vi "UHR-Fleezers Control (host) - Avogadro v1.vi"() -> ()   [LabVIEW 2014] (continued)
          n911 = property on="Base N trap periods" class="DigNum (strict)"("Val(Sgnl)"=w1415) -> ()  [unwired: 2 in, 2 out]
        }
      }
    }
    frame #4 {
      # "Set FIFO size and run FPGA"
      n912 = local read "FPGA error out"() -> (w1417:errorcluster)
      n913 = xnode "Invoke Method"("FPGA VI Reference In"=w1418, "error in"=w1417, "Requested Depth"="Trap AI FIFO Depth") -> ("FPGA VI Reference Out"=w1422:T41, "error out"=w1423:errorcluster)  [unwired: 1 out]
      n914 = xnode "Invoke Method"("FPGA VI Reference In"=w1422, "error in"=w1423, "Requested Depth"="Trap Position FIFO Depth") -> ("FPGA VI Reference Out"=w1420:T41, "error out"=w1419:errorcluster)  [unwired: 1 out]
      n915 = xnode "Invoke Method"("FPGA VI Reference In"=w1420, "error in"=w1419) -> ("error out"=w1416:errorcluster)  [unwired: 1 in, 1 out]
      n916 = local write "FPGA error out"(w1416) -> ()
    }
    frame #5 {
      # "Adjust FPGA timing loop phases"
      n917 = flat-sequence "Initial FPGA Loop Relative Phase Adjustment" {
        tunnel: "Initial Phase Adjustment (AI1)" -> [w1457]
        tunnel: "Initial Phase Adjustment (GI)" -> [w1456]
        tunnel: "Initial Phase Adj. (MCL)" -> [w1455]
        tunnel: [w1458] -> w1442
        tunnel: [w1454] -> w1441
        tunnel: "Initial Phase Adjustment (APD Acq)" -> [w1453]
        tunnel: "Initial Phase Adjustment (APD 1 Gate)" -> [w1452]
        tunnel: "Initial Phase Adjustment (Green FB)" -> [w1451]
        tunnel: "Initial Phase Adjustment (GI) 2" -> [w1450]
        tunnel: "Initial Phase Adjustment (APD 2 Gate)" -> [w1449]
        tunnel: "Initial Phase Adjustment (RI)" -> [w1448]
        tunnel: "Initial Phase Adjustment (BI DO)" -> [w1447]
        tunnel: "Initial Phase Adjustment (BI AO)" -> [w1446]
        tunnel: "Initial Phase Adjustment (APD 3 Gate)" -> [w1445]
        tunnel: w1427 -> [w1444]
        tunnel: w1442 -> [w1460]
        tunnel: [w1461] -> w1440
        tunnel: w1441 -> [w1461]
        tunnel: [w1460] -> w1439
        tunnel: w1440 -> [w1465]
        tunnel: w1439 -> [w1464]
        tunnel: [w1462] -> w1426
        frame #0 {
          n918 = local read "FPGA error out"() -> (w1443:errorcluster)
          n919 = xnode "Read/Write Control"("FPGA VI Reference In"=w1444, "error in"=w1443, "Phase count adjustment"=w1457, "Phase count adjustment (GI)"=w1456, "Phase count adjustment (MCL)"=w1455, "Phase Count Adjustment (APD Acq)"=w1453, "Phase count adjustment (APD 1 Gate)"=w1452, "Phase count adjustment (APD 2 Gate)"=w1449, "Phase count adjustment (Green FB)"=w1451, "Phase count adjustment (GI) 2"=w1450, "Phase count adjustment (RI)"=w1448, "Phase count adjustment (BI AO)"=w1446, "Phase count adjustment (BI D)"=w1447, "Phase count adjustment (APD 3 Gate)"=w1445) -> ("FPGA VI Reference Out"=w1454:T41, "error out"=w1458:errorcluster)
        }
        frame #1 {
          n920 = Wait (ms)(milliseconds to wait=u32 100) -> ()  [unwired: 1 out]
        }
        frame #2 {
          w1463 = TRUE
          n921 = xnode "Read/Write Control"("FPGA VI Reference In"=w1465, "error in"=w1464, "+ phase"=w1463, "+ phase (GI)"=w1463, "+ phase (MCL)"=w1463, "+ phase (APD Acq)"=w1463, "+ phase (APD 1 Gate)"=w1463, "+ phase (APD 2 Gate)"=w1463, "+ phase (Green FB)"=w1463, "+ phase (GI) 2"=w1463, "+ phase (RI)"=w1463, "+ phase (BI AO)"=w1463, "+ phase (BI D)"=w1463, "+ phase (APD 3 Gate)"=w1463) -> ("error out"=w1462:errorcluster)  [unwired: 1 out]
        }
      }
      n922 = local write "FPGA error out"(w1426) -> ()
    }
    frame #6 {
      w1479 = 6.0  # clock mult.
      w1478 = 49152000.0  # TCXO frequ.
      w1483 = 6.0  # clock mult.
      w1484 = 49152000.0  # TCXO frequ.
      # "Added by ronen - definition of \nlimit frequencies when using dynamic feedback"
      # "Initialize trap RF synth board and set initial frequencies and amplitudes"
      n923 = local read "FPGA error out"() -> (w1493:errorcluster)
      n924 = call "Initialize RF boards - interlace 3.vi"("error in"=w1493, "FPGA VI Reference In"=w1494) -> ("error out"=w1495:errorcluster, "FPGA VI Reference Out"=w1515:T41)
      n925 = call "set RF board frequency - interlace.vi"("Board 2 Frequency Limits"=w1490, "Board 1 Frequency Limits"=w1471, "error in"=w1495, "FPGA VI Reference In"=w1515, "Board 2 Frequency 3 (MHz)"="BD 2 Frequency 3 (MHz)", "Board 1 Frequency 3 (MHz)"="BD 1 Frequency 3 (MHz)", "Board 2 Frequency 2 (MHz)"="BD 2 Frequency 2 (MHz)", "Board 2 Frequency 1 (MHz)"="BD 2 Frequency 1 (MHz)", "Board 1 Frequency 2 (MHz)"="BD 1 Frequency 2 (MHz)", "Board 1 Frequency 1  (MHz)"="BD 1 Frequency 1 (MHz)") -> ("error out"=w1498:errorcluster, "FPGA VI Reference Out"=w1470:T41)
      n926 = Unbundle By Name(w1471) -> ("Maximum"=w1481:dbl, "Minimum"=w1472:dbl)
      n927 = call "set RF board amplitude - interlace.vi"("Board 2 Amplitude Limits"=w1492, "Board 1 Amplitude Limits"=w1491, "error in"=w1498, "FPGA VI Reference In"=w1470, "Board 2 Amplitude 3 (%)"="BD 2 Amplitude 3 (%)", "Board 1 Amplitude 3 (%)"="BD 1 Amplitude 3 (%)", "Board 2 Amplitude 2 (%)"="BD 2 Amplitude 2 (%)", "Board 2 Amplitude 1 (%)"="BD 2 Amplitude 1 (%)", "Board 1 Amplitude 2 (%)"="BD 1 Amplitude 2 (%)", "Board 1 Amplitude 1 (%)"="BD 1 Amplitude 1 (%)") -> ("error out"=w1467:errorcluster)  [unwired: 1 out]
      n928 = Multiply(x=w1472, y=1000000.0) -> (x*y=w1476:dbl)
      n929 = Multiply(x=w1481, y=1000000.0) -> (x*y=w1486:dbl)
      n930 = Scale By Power Of 2(n=48, x=w1476) -> (x*2^n=w1474:dbl)
      n931 = Subtract(x="BD 1 Frequency 1 (MHz)", y="BD 1 Frequency 2 (MHz)") -> (x-y=w1505:dbl)
      n932 = Subtract(x="BD 2 Frequency 1 (MHz)", y="BD 2 Frequency 2 (MHz)") -> (x-y=w1506:dbl)
      n933 = Scale By Power Of 2(n=48, x=w1486) -> (x*2^n=w1488:dbl)
      n934 = Multiply(x=w1478, y=w1479) -> (x*y=w1480:dbl)
      n935 = Multiply(x=w1484, y=w1483) -> (x*y=w1482:dbl)
      n936 = Square(x=w1506) -> (x^2=w1508:dbl)
      n937 = Square(x=w1505) -> (x^2=w1507:dbl)
      n938 = Divide(x=w1474, y=w1480) -> (x/y=w1475:dbl)
      n939 = Divide(x=w1488, y=w1482) -> (x/y=w1487:dbl)
      n940 = Add(x=w1507, y=w1508) -> (x+y=w1509:dbl)
      n941 = To Unsigned Quad Integer(1:w1475) -> (0:w1468:u64)
      n942 = To Unsigned Quad Integer(1:w1487) -> (0:w1469:u64)
      n943 = Square Root(x=w1509) -> (sqrt(x)=w1510:dbl)
      n944 = local write "Trap Delta (MHz)"(w1510) -> ()
      n945 = xnode "Read/Write Control"("FPGA VI Reference In"=w1470, "error in"=w1467, "FB Max Frequency"=w1469, "FB Min frequency"=w1468) -> ("error out"=w1466:errorcluster)  [unwired: 1 out]
      n946 = local write "FPGA error out"(w1466) -> ()
    }
    frame #7 {
      n947 = local read "FPGA error out"() -> (w1517:errorcluster)
      n948 = flat-sequence {
        tunnel: [w1531] -> w1522
        tunnel: [w1530] -> w1521
        tunnel: w1518 -> [w1524]
        tunnel: w1517 -> [w1523]
        tunnel: [w1535] -> w1520
        tunnel: w1522 -> [w1535]
        tunnel: [w1534] -> w1519
        tunnel: w1521 -> [w1534]
        tunnel: w1520 -> [w1543]
        tunnel: w1519 -> [w1542]
        tunnel: [w1537] -> w1516
        frame #0 {
          n949 = xnode "Read/Write Control"("FPGA VI Reference In"=w1524, "error in"=w1523, "Direct RF Box  Communication"=FALSE) -> ("FPGA VI Reference Out"=w1531:T41, "error out"=w1530:errorcluster)
          n950 = local read "Trap 1 (ON/OFF)"() -> (w1525:bool)
          n951 = local write "Saving..."(FALSE ("Saving Data")) -> ()
          n952 = local write "Stop All"(FALSE ("Stop All")) -> ()
          n953 = local write "Index"(1.0 ("Index")) -> ()
          n954 = property on="Trap 1 ON" class="Bool (strict)"("Value"=w1525) -> ()  [unwired: 2 in, 2 out]
          "Manipulating Trap" <- FALSE ("Manipulating Trap")
        }
        frame #1 {
          n955 = local read "Trap 2 (ON/OFF)"() -> (w1533:bool)
          n956 = Wait (ms)(milliseconds to wait=u32 10) -> ()  [unwired: 1 out]
          n957 = property on="Trap 2 ON" class="Bool (strict)"("Val(Sgnl)"=w1533) -> ()  [unwired: 2 in, 2 out]
        }
        frame #2 {
          n958 = local read "Scan Range (nm)"() -> (w1538:dbl)
          n959 = xnode "Read/Write Control"("FPGA VI Reference In"=w1543, "error in"=w1542, "FPGA Controls  RF Box"=TRUE ("Direct RF Box  Communication")) -> ("error out"=w1537:errorcluster)  [unwired: 1 out]
          n960 = call "Update messages.vi"("Message to add"="UHR-Fleezers ready.", "Old message string"="") -> ("New message string"=w1541:string)
          n961 = local write "Messages"(w1541) -> ()
          n962 = property on="Scan Range (nm)" class="DigNum (strict)"("Val(Sgnl)"=w1538) -> ()  [unwired: 2 in, 2 out]
        }
      }
      n963 = local write "FPGA error out"(w1516) -> ()
    }
    frame #8 {
      w1577 = u32 0
      w1583 = cluster{u32, u32} {16777238, 16777238}
      w1578 = 0.0
      # "Initialize valves"
      # "Cursor control of trap\n3"
      # "Graph of positions and displacements in 2D"
      n964 = call "start_stage_trackball.vi"("Enum"=T38."Trackball XY", "Stage Controller port"=w1547) -> ("error out"=w1545:errorcluster)  [unwired: 1 in, 1 out]
      n965 = property on="Stage Control Serial Error" class="Clust (strict)"("Val(Sgnl)"=w1545) -> ()  [unwired: 2 in, 2 out]
      n966 = control-ref of="Positions \nand displacements"() -> (w1567:refnum<vi>)
      n967 = control-ref of="Piezo trap cursor control"() -> (w1579:refnum<vi>)
      n968 = property class="XYGraph (strict)"(reference=w1567, "XScale.Maximum"=6500.0, "XScale.Minimum"=-400.0, "YScale.Maximum"=400.0, "YScale.Minimum"=-3200.0, "Frame Color"=u32 9868950) -> (reference out=w1548:refnum<vi>)  [unwired: 1 in, 1 out]
      n969 = property class="XYGraph (strict)"(reference=w1548, "Active Plot"=0, "Plot.Plot Color"=u32 16711680, "Plot.Point Style"=2, "Plot.Line Width"=5, "Plot.Plot Interpolation"=0) -> (reference out=w1554:refnum<vi>)  [unwired: 1 in, 1 out]
      n970 = property class="XYGraph (strict)"(reference=w1579, "XScale.Maximum"=10.0, "XScale.Minimum"=w1578, "YScale.Maximum"=w1578, "YScale.Minimum"=-10.0, "Plot Area Colors"=w1583, "Frame Color"=u32 9868950, "XScale.GridColors"=w1583, "YScale.GridColors"=w1583, "Cursor.Cursor Color"=u32 16711680, "Active Cursor"=w1577, "Cursor.CursorMode"=w1577) -> ()  [unwired: 1 in, 2 out]
      n971 = property class="XYGraph (strict)"(reference=w1554, "Active Plot"=1, "Plot.Plot Color"=u32 16711680, "Plot.Point Style"=2, "Plot.Line Width"=5, "Plot.Plot Interpolation"=0) -> (reference out=w1555:refnum<vi>)  [unwired: 1 in, 1 out]
      n972 = property class="XYGraph (strict)"(reference=w1555, "Active Plot"=2, "Plot.Plot Color"=u32 16711680, "Plot.Point Style"=2, "Plot.Line Width"=5, "Plot.Plot Interpolation"=0) -> ()  [unwired: 1 in, 2 out]
      n973 = call "hamilton_controller.vi"("VISA resource name in"="Visa resource for valves", "action"=T42."CONNECT") -> ("error out"=w1576:errorcluster, "VISA resource name out"=w1573:refnum<visa-resource-name>)  [unwired: 8 in]
      n974 = call "hamilton_controller.vi"("VISA resource name in"=w1573, "error in"=w1576, "action"=T42."INITIALIZE VALVES") -> ("error out"=w1585:errorcluster)  [unwired: 7 in, 1 out]
    }
    frame #9 {
      # "Wait 5 s for all the event loops still being executed to finish."
      n975 = Wait (ms)(milliseconds to wait=u32 5000) -> ()  [unwired: 1 out]
      n976 = local read "FPGA error out"() -> (w1587:errorcluster)
    }
  }
  n977 = node-c288() -> (w34:T35)  [unwired: 4 out]
  n978 = disable-structure shown="Disabled" {
    frame Disabled {
      n979 = while "Duncan's play event loop" {
        stop <- w1591 stop-if-true
        n980 = Create User Event(user event datatype=TRUE ("Boolean")) -> (user event=w1592:refnum<user-event>)  [unwired: 1 in, 1 out]
        n981 = Create User Event(user event datatype=TRUE ("Boolean")) -> (user event=w1598:refnum<user-event>)  [unwired: 1 in, 1 out]
        n982 = global write "Global for fluorescence simulation mean (30 samples), (power series).vi" "Red Signal"(w1592) -> ()
        n983 = global write "Global for fluorescence simulation mean (30 samples), (power series).vi" "Green Signal"(w1598) -> ()
        n984 = register-events(w1598, w1592) -> (reference out=w1597:refnum<event-registration>)  [unwired: 2 in, 1 out]
        n985 = event shown="[1] \"Start assembly line\": Value Change" {
          selector: w1597 -> [_ _ _ _]
          dyn-events: _ -> [_ _ _ _]
          timeout: 100 -> [_ _ _ _]
          event Timeout {
            n986 = event-data() -> ()  [unwired: 1 in, 2 out]
          }
          event "Start assembly line": Value Change {
            n987 = event-data() -> ("OldVal"=w1600:bool)  [unwired: 1 in, 4 out]
            n988 = case shown="True" w1600 {
              selector: w1600 -> [_ w1601]
              frame False {
              }
              frame True {
                n989 = property on="Move to Position 3" class="Bool (strict)"("Val(Sgnl)"=w1601) -> ()  [unwired: 2 in, 2 out]
                n990 = case shown="1" "Numeric" {
                  frame 0, Default {
                  }
                  frame 1 {
                    n991 = property on="Green Laser ON" class="Bool (strict)"("Val(Sgnl)"=TRUE ("Value (Signaling)")) -> ()  [unwired: 2 in, 2 out]
                  }
                  frame 2 {
                    n992 = property on="Red Laser ON" class="Bool (strict)"("Val(Sgnl)"=TRUE) -> ()  [unwired: 2 in, 2 out]
                  }
                }
              }
            }
          }
          event User Event {
            n993 = event-data() -> ("Boolean"=w1605:bool)  [unwired: 1 in, 3 out]
            "Green Fluorophore" <- w1605
            n994 = property on="Start assembly line" class="Bool"("Val(Sgnl)"=w1605) -> ()  [unwired: 2 in, 2 out]
          }
          event User Event {
            n995 = event-data() -> ("Boolean"=w1606:bool)  [unwired: 1 in, 3 out]
            "Red Fluorophore" <- w1606
            n996 = property on="Start assembly line" class="Bool"("Val(Sgnl)"=w1606) -> ()  [unwired: 2 in, 2 out]
          }
        }
        n997 = property on="Get Fluorophore" class="Bool (strict)"("Val(Sgnl)"="Get Fluorophore") -> ()  [unwired: 2 in, 2 out]
        n998 = Wait (ms)(milliseconds to wait=u32 100) -> ()  [unwired: 1 out]
        n999 = local read "Stop All"() -> (w1590:bool)
        n1000 = Or(x=w1590, y="stop") -> (x .or. y?=w1591:bool)
      }
    }
    frame Enabled {
    }
  }
  n1001 = timed-loop "Rough control of MCL mirror stage (debugging)" {
    tunnel: [w1609] -> w74
    timing: w34 -> [_]
    timing-out: [_] -> w33
    tunnel: w25 -> [w1607]
    stop <- w1609 stop-if-true
    n1002 = node-c288() -> ()  [unwired: 2 out]
    n1003 = case shown="1" "MCL Mode" {
      tunnel: w1607 -> [_ w1612 w1659]
      frame 0, Default {
      }
      frame 1 {
        n1004 = node-c288() -> (w1614:T35)  [unwired: 4 out]
        n1005 = timed-loop "Oscillate MCL mirror" {
          timing: w1614 -> [_]
          timing-out: [_] -> w1613
          tunnel: w1612 -> [w1615]
          i -> [w1653]
          stop <- w1616 stop-if-true
          n1006 = node-c288() -> (w1652:i64)  [unwired: 1 out]
          n1007 = Multiply(x="AO1", y=32767.0) -> (x*y=w1648:dbl)
          n1008 = Multiply(x="AO2", y=32767.0) -> (x*y=w1643:dbl)
          n1009 = Divide(x=w1648, y=10.0) -> (x/y=w1649:dbl)
          n1010 = Divide(x=w1643, y=10.0) -> (x/y=w1644:dbl)
          n1011 = To Word Integer(number=w1649) -> (16bit integer=w1641:i16)
          n1012 = To Word Integer(number=w1644) -> (16bit integer=w1640:i16)
          n1013 = Divide(x=w1652, y=i64 1000) -> (x/y=w1623:dbl)
          n1014 = Multiply(x=w1623, y=w1653) -> (x*y=w1634:dbl)
          n1015 = Multiply(x="Osc. freq. (Hz) 2", y=6.283185307179586) -> (x*y=w1635:dbl)
          n1016 = Multiply(x=w1635, y=w1634) -> (x*y=w1633:dbl)
          n1017 = Sine(x=w1633) -> (sin(x)=w1632:dbl)
          n1018 = Multiply(x=w1632, y="Osc. amp. (V)") -> (x*y=w1630:dbl)
          n1019 = Add(x=w1630, y="Osc. center (V)") -> (x+y=w1628:dbl)
          n1020 = Divide(x=w1628, y=10.0) -> (x/y=w1626:dbl)
          n1021 = Multiply(x=w1626, y=32767.0) -> (x*y=w1621:dbl)
          n1022 = Select(t=w1621, s="Scan axis", f=w1641) -> (s? t:f=w1639:dbl)
          n1023 = Select(t=w1640, s="Scan axis", f=w1621) -> (s? t:f=w1638:dbl)
          n1024 = local read "MCL Mode"() -> (w1620:u16)
          n1025 = Not Equal?(x=w1620, y=u16 1) -> (x != y?=w1617:bool)
          n1026 = local read "Stop All"() -> (w1618:bool)
          n1027 = xnode "Read/Write Control"("FPGA VI Reference In"=w1615, "AO1 (Y)"=w1639, "AO2 (X)"=w1638) -> ()  [unwired: 1 in, 2 out]
          n1028 = Compound Arithmetic op=OR(w1618, w1617) -> (w1616:bool)
          n1029 = node-c288() -> ()  [unwired: 2 out]
        }
        n1030 = node-c288(w1613) -> ()  [unwired: 1 out]
      }
      frame 2 {
        n1031 = case shown="True" "Start Scan" {
          tunnel: w1659 -> [_ w1661]
          frame False {
          }
          frame True {
            n1032 = Subtract(x="End (V)", y="Begin (V)") -> (x-y=w1668:dbl)
            n1033 = Decrement(x="N Points") -> (x-1=w1667:dbl)
            n1034 = Divide(x=w1668, y=w1667) -> (x/y=w1665:dbl)
            n1035 = for {
              N: "N Points" -> [_]
              tunnel: "Begin (V)" -> [w1684]
              tunnel: [w1676] -> w1671 mode=indexing
              tunnel: w1665 -> [w1675]
              tunnel: [w1673] -> w1664 mode=indexing
              tunnel: w1661 -> [w1672]
              i -> [w1683]
              n1036 = Multiply(x=w1675, y=w1683) -> (x*y=w1682:dbl)
              n1037 = Add(x=w1684, y=w1682) -> (x+y=w1679:dbl)
              n1038 = local read "Scan axis"() -> (w1674:bool)
              n1039 = local read "AO1"() -> (w1681:dbl)
              n1040 = local read "AO2"() -> (w1680:dbl)
              n1041 = Select(t=w1679, s=w1674, f=w1681) -> (s? t:f=w1678:dbl)
              n1042 = Select(t=w1680, s=w1674, f=w1679) -> (s? t:f=w1677:dbl)
              n1043 = flat-sequence {
                tunnel: w1678 -> [w1688]
                tunnel: w1677 -> [w1687]
                tunnel: w1672 -> [w1685]
                tunnel: [w1698] -> w1676
                tunnel: [w1697] -> w1673
                frame #0 {
                  w1691 = 10.0 ("y")
                  w1686 = 32767.0 ("y")
                  n1044 = Multiply(x=w1688, y=w1686) -> (x*y=w1694:dbl)
                  n1045 = Multiply(x=w1687, y=w1686) -> (x*y=w1692:dbl)
                  n1046 = Divide(x=w1694, y=w1691) -> (x/y=w1695:dbl)
                  n1047 = Divide(x=w1692, y=w1691) -> (x/y=w1693:dbl)
                  n1048 = To Word Integer(number=w1695) -> (16bit integer=w1689:i16)
                  n1049 = To Word Integer(number=w1693) -> (16bit integer=w1690:i16)
                  n1050 = xnode "Read/Write Control"("FPGA VI Reference In"=w1685, "AO1 (Y)"=w1689, "AO2 (X)"=w1690) -> ()  [unwired: 1 in, 2 out]
                }
                frame #1 {
                  n1051 = Wait (ms)(milliseconds to wait="DAQ Delay (ms)") -> ()  [unwired: 1 out]
                }
                frame #2 {
                  n1052 = local read "Slow mean"() -> (w1698:dbl)
                  n1053 = local read "Sigma"() -> (w1697:dbl)
                }
              }
            }
            n1054 = Bundle("Begin (V)"="Begin (V)", w1665, w1671) -> (→"MCL Scan":cluster{"Begin (V)":dbl, dbl, dbl[]})  [unwired: 1 out]
            n1055 = Bundle("Begin (V)"="Begin (V)", w1665, w1664) -> (→"MCL Scan 2":cluster{"Begin (V)":dbl, dbl, dbl[]})  [unwired: 1 out]
          }
        }
      }
    }
    n1056 = local read "Stop All"() -> (w1609:bool)
    n1057 = node-c288() -> ()  [unwired: 2 out]
  }
  n1058 = node-c288(2 ("Processor")) -> (w65:T35)  [unwired: 3 out]
  n1059 = timed-loop "Basic control parameters (all FPGA settings, other basic controls)" {
    shift-right: [w1706] -> _
    shift-left: errorcluster {"status"=FALSE, "code"=0, "source"=""} ("error out") -> [_]
    tunnel: [w1705] -> _
    timing: w65 -> [_]
    timing-out: [_] -> w64
    tunnel: w47 -> [w1704]
    tunnel: w43 -> [w1703]
    tunnel: w42 -> [w1702]
    tunnel: w41 -> [w1701]
    tunnel: w40 -> [w1700]
    tunnel: w25 -> [w1699]
    stop <- w1705 stop-if-true
    n1060 = node-c288() -> ()  [unwired: 2 out]
    n1061 = event shown="[13] \"Load parameters\": Value Change" {
      selector: _ -> [_ _ _ _ _ _ _ _ _ _ _ _ _ _ _ _ _ _ _ _ _ _ _ _ _ _ _ _ _ _ _ _ _ _ _ _ _ _ _ _ _ _ _ _ _ _ _ _ _ _ _ _ _ _ _ _ _ _ _ _ _ _ _ _ _ _ _ _ _ _ _ _ _ _ _ _ _ _ _ _ _ _ _ _ _ _]
      dyn-events: _ -> [_ _ _ _ _ _ _ _ _ _ _ _ _ _ _ _ _ _ _ _ _ _ _ _ _ _ _ _ _ _ _ _ _ _ _ _ _ _ _ _ _ _ _ _ _ _ _ _ _ _ _ _ _ _ _ _ _ _ _ _ _ _ _ _ _ _ _ _ _ _ _ _ _ _ _ _ _ _ _ _ _ _ _ _ _ _]
      timeout: _ -> [_ _ _ _ _ _ _ _ _ _ _ _ _ _ _ _ _ _ _ _ _ _ _ _ _ _ _ _ _ _ _ _ _ _ _ _ _ _ _ _ _ _ _ _ _ _ _ _ _ _ _ _ _ _ _ _ _ _ _ _ _ _ _ _ _ _ _ _ _ _ _ _ _ _ _ _ _ _ _ _ _ _ _ _ _ _]
      tunnel: [w1746 _ _ _ w1773 _ _ _ _ _ _ _ w1879 _ _ w1966 w1968 w1975 w1977 w2047 _ w2089 w2115 w2143 w2168 w2195 w2221 w2250 _ w2255 w2349 w2353 w2390 _ w2475 w2478 w2481 w2491 w2494 _ w2501 _ _ _ _ _ _ _ _ _ _ _ _ _ _ _ _ _ _ _ w2996 _ _ _ _ w3033 _ _ _ _ _ _ _ _ _ _ _ _ _ _ _ _ _ _ _ _] -> w1706
      tunnel: [_ _ _ _ _ _ _ _ _ _ w1858 _ _ _ _ _ _ _ _ _ _ _ _ _ _ _ _ _ _ _ _ _ _ _ _ _ _ _ _ _ _ _ _ _ _ _ _ _ _ _ _ _ _ _ _ _ _ _ _ _ _ _ _ _ _ _ _ _ _ _ _ _ _ _ _ _ _ _ _ _ _ _ _ _ _ _] -> w1705
      tunnel: [_ _ _ _ _ _ _ _ "Round T1 X" _ _ _ _ _ _ _ _ _ _ _ _ _ _ _ _ _ _ _ _ _ _ _ _ _ _ _ _ _ _ _ _ _ _ _ _ _ _ _ _ _ _ _ _ _ _ _ _ _ _ _ _ _ _ _ _ _ _ _ _ _ _ _ _ _ _ _ _ _ _ _ _ _ _ _ _ _] -> _
      tunnel: [_ _ _ "Adjust Scale\nto Mean" _ _ _ _ _ _ _ _ _ _ _ _ _ _ _ _ _ _ _ _ _ _ _ _ _ "Test ttrig" _ _ _ _ _ _ _ _ _ _ _ _ _ _ _ _ _ _ _ _ w2743 w2807 w2854 w2903 _ _ _ _ _ _ _ _ _ _ _ _ _ _ _ _ _ _ _ _ _ _ _ _ _ _ _ _ _ _ _ _] -> _
      tunnel: [_ _ _ _ _ _ _ _ _ "Round T2 X" _ "Delayed Interlace Start" _ _ _ _ _ _ _ _ _ _ _ _ _ _ _ _ _ _ _ _ _ _ _ _ _ _ _ _ _ _ _ _ _ _ _ _ _ _ _ _ _ _ _ _ _ _ _ _ _ _ _ _ _ _ _ _ _ _ _ _ _ _ _ _ _ _ _ _ _ _ _ _ _ _] -> _
      tunnel: w1704 -> [_ _ _ _ _ _ _ _ _ _ _ _ _ _ _ _ _ _ _ _ _ _ _ _ _ _ _ _ _ _ _ _ _ _ _ _ _ _ _ _ _ _ _ _ _ _ w2713 w2721 w2728 w2734 w2742 _ _ w2902 _ _ _ _ _ _ _ _ _ _ _ _ _ _ _ _ _ _ _ _ _ _ _ _ _ _ _ _ _ _ _ _]
      tunnel: w1703 -> [_ _ _ _ _ _ _ _ _ _ _ _ _ _ _ _ _ _ _ _ _ _ _ _ _ _ _ _ _ _ _ _ _ _ _ _ _ _ _ _ _ _ _ _ w2600 _ _ _ _ _ _ w2806 _ _ w2909 _ w2921 _ w2937 _ _ _ _ _ _ _ _ _ _ _ _ _ _ _ _ _ _ _ _ _ _ _ _ _ _ _]
      tunnel: w1702 -> [_ _ _ _ _ _ _ _ _ _ _ _ _ _ _ _ _ _ _ _ _ _ _ _ _ _ _ _ _ _ _ _ _ _ _ _ _ _ _ _ _ _ _ _ _ _ _ _ _ _ _ _ _ _ _ _ _ _ _ _ _ _ _ _ _ _ _ _ _ _ _ _ _ _ _ _ _ _ _ _ _ _ _ _ _ _]
      tunnel: w1701 -> [_ _ _ _ _ _ _ _ _ _ _ _ _ _ _ _ _ _ _ _ _ _ _ _ _ _ _ _ _ _ _ _ _ _ _ _ _ _ _ _ _ w2512 _ _ _ _ _ _ _ _ _ _ w2853 _ _ w2915 _ w2929 _ w2963 _ _ _ _ _ _ _ _ _ _ _ _ _ _ _ _ _ _ _ _ _ _ _ _ _ _]
      tunnel: w1700 -> [_ _ _ _ _ _ _ _ _ _ _ _ _ _ _ _ _ _ _ _ _ _ _ _ _ _ _ _ _ _ _ _ _ _ _ _ _ _ _ _ _ _ _ _ _ _ _ _ _ _ _ _ _ _ _ _ _ _ _ _ _ _ _ _ _ _ _ _ _ _ _ _ _ _ _ _ _ _ _ _ _ _ _ _ _ _]
      tunnel: w1699 -> [w1709 _ _ _ w1772 _ w1798 _ _ _ _ _ w1870 _ _ w1950 w1967 w1974 w1976 w2012 _ w2078 w2113 w2125 w2150 w2178 w2198 w2226 w2251 w2253 w2257 w2350 w2354 _ w2472 w2476 w2479 w2489 w2492 _ w2500 _ _ _ _ _ _ _ _ _ _ _ _ _ _ _ _ _ _ _ w2989 _ w3010 _ w3017 w3032 _ w3039 w3066 w3073 w3089 w3097 _ w3108 _ w3152 _ _ w3206 w3237 w3241 w3249 _ w3313 w3323 w3342]
      tunnel: [_ _ _ _ _ _ _ _ _ _ w1857 _ _ _ _ _ _ _ _ _ _ _ _ _ _ _ _ _ _ _ _ _ _ _ _ _ _ _ _ _ _ _ w2592 w2596 _ _ _ _ _ _ _ _ _ _ _ _ _ _ _ _ _ _ _ _ _ _ _ _ _ _ _ _ _ _ _ _ _ _ _ _ _ _ _ _ _ _] -> _
      event "AI Count (ticks)", "Sets to FIFO (Traps)", "Save ave N", "FPGA Ave.", "# Samples/channel", "N sets to save": Value Change {
        # "RG 18-01-16 Increased amount of elements to read for trap position, to add x and y for piezo trap"
        # "So that if 'Save ave N' is updated, the AOD scanning code updates too."
        n1062 = event-data() -> ()  [unwired: 6 out]
        n1063 = local read "AI Count (ticks)"() -> (w1730:u16)
        n1064 = Divide(x=40000000.0, y=w1730) -> (x/y=w1722:dbl)
        "AI rate (Hz)" <- w1722
        "Ave. Rate (Hz)" <- w1722
        n1065 = Reciprocal(x=w1722) -> (1/x=→"Ave. Period (s)":dbl)
        n1066 = Unbundle By Name("Sets to FIFO (Traps)") -> ("Set 1"=w1713:bool, "Set 2"=w1712:bool, "Set 3"=w1711:bool)
        n1067 = Divide(x=w1722, y="N Acq Sets (Traps + Fl.)") -> (x/y=w1743:dbl)
        "Data Rate (Hz)" <- w1743
        n1068 = Reciprocal(x=w1743) -> (1/x=→"Data Period (s)":dbl)
        n1069 = Boolean To (0,1)(Boolean="Sets to FIFO (Traps)") -> (0, 1=w1738:cluster{"Set 1":i16, "Set 2":i16, "Set 3":i16})
        n1070 = xnode "Read/Write Control"("FPGA VI Reference In"=w1709, "ai count"=w1730, "Set 1"=w1713, "Set 2"=w1712, "Set 3"=w1711, "N of AI1 Int Acq Sets"="N Acq Sets (Traps + Fl.)") -> ("error out"=w1746:errorcluster)  [unwired: 1 in, 1 out]
        n1071 = Cluster To Array(cluster=w1738) -> (array=w1737:i16[])
        n1072 = local read "Save ave N"() -> (w1742:dbl)
        n1073 = To Unsigned Long Integer(number=w1737) -> (unsigned 32bit integer=w1719:u32[])
        n1074 = local read "Scan steps (AOD)"() -> (w1739:u64)
        n1075 = Multiply(x=w1730, y="N Acq Sets (Traps + Fl.)") -> (x*y=w1728:u16)
        n1076 = Add Array Elements(numeric array=w1719) -> (sum=w1731:u32)
        "Trap Sets" <- w1731
        n1077 = Divide(x=w1743, y=w1742) -> (x/y=w1741:dbl)
        "Save Data Rate (Hz)" <- w1741
        n1078 = Reciprocal(x=w1741) -> (1/x=→"Save Data Period (s)":dbl)
        n1079 = property on="Scan steps (AOD)" class="DigNum (strict)"("Val(Sgnl)"=w1739) -> ()  [unwired: 2 in, 2 out]
        n1080 = Multiply(x=w1728, y="# Samples/trap") -> (x*y=w1726:u32)
        "Counts/DMA" <- w1726
        n1081 = property on="Trap Disp. Downsample" class="DigNum (strict)"("Maximum"="# Samples/trap") -> ()  [unwired: 2 in, 2 out]
        n1082 = Multiply(x=w1731, y="# Samples/trap") -> (x*y=w1720:u32)
        "# Samples/channel" <- w1720
        n1083 = Multiply(x=w1720, y=u32 8) -> (x*y=→"Trap AI Elements/DMA read":u32)
        n1084 = local read "APD Int. Count"() -> (w1727:u32)
        n1085 = Multiply(x=w1720, y=u32 5) -> (x*y=→"Trap Pos Elements/DMA read":u32)
        n1086 = Divide(x=w1726, y=w1727) -> (x/y=w1717:dbl)
        "APD Samples/FIFO Acq." <- w1717
        n1087 = Divide(x=w1726, y=40000000.0) -> (x/y=w1724:dbl)
        "DMA Update Period (s)" <- w1724
        n1088 = local read "Number of APDs"() -> (w1710:u8)
        n1089 = Multiply(x=w1710, y=w1717) -> (x*y=→"APD Elements/DMA read":dbl)
        n1090 = property on="APD Disp. Downsample" class="DigNum (strict)"("Maximum"=w1717) -> ()  [unwired: 2 in, 2 out]
        n1091 = local read "N sets to save"() -> (w1736:u32)
        n1092 = Multiply(x=w1724, y=w1736) -> (x*y=→"Total Time (s) 2":dbl)
        "FPGA Averaging" <- FALSE ("FPGA Averaging")
      }
      event "Remove Offset": Value Change {
        n1093 = event-data() -> ()  [unwired: 7 out]
        n1094 = local write "Remove Offset"(FALSE ("Remove Offset")) -> ()
        n1095 = local read "Bead Mean (nm)"() -> (w1748:dbl)
        n1096 = local read "Offset (nm)"() -> (w1749:dbl)
        n1097 = Add(x=w1748, y=w1749) -> (x+y=w1747:dbl)
        n1098 = local write "Offset (nm)"(w1747) -> ()
      }
      event "Detector Type": Value Change {
        n1099 = event-data() -> ()  [unwired: 7 out]
        n1100 = local read "AI labels"() -> (w1753:string[])
        n1101 = property on="High Res. Display" class="Ring (strict)"("Strings []"=w1753) -> ()  [unwired: 2 in, 2 out]
        n1102 = Build Array (concatenate)(w1753, "none") -> (w1754:string[])
        n1103 = property on="FFT 1 Choice 1" class="Ring (strict)"("Strings []"=w1754) -> ()  [unwired: 2 in, 2 out]
        n1104 = property on="FFT 1 Choice 2" class="Ring (strict)"("Strings []"=w1754) -> ()  [unwired: 2 in, 2 out]
        n1105 = property on="FFT 2 Choice 1" class="Ring (strict)"("Strings []"=w1754) -> ()  [unwired: 2 in, 2 out]
        n1106 = property on="FFT 2 Choice 2" class="Ring (strict)"("Strings []"=w1754) -> ()  [unwired: 2 in, 2 out]
        n1107 = Bundle("APD 1", "APD 2", "APD 3") -> (w1757:cluster{string, string, string})  [unwired: 1 out]
        n1108 = Cluster To Array(cluster=w1757) -> (array=w1755:string[])
        n1109 = Build Array (concatenate)(w1755, w1754) -> (w1759:string[])
        n1110 = Array Size(array=w1759) -> (size(s)=w1751:i32)
        n1111 = property on="Signals to Plot" class="LstBox (strict)"("Item Names"=w1759) -> ()  [unwired: 2 in, 2 out]
        n1112 = property on="Signals to Plot" class="LstBox (strict)"("Number of Rows"=w1751) -> ()  [unwired: 2 in, 2 out]
        n1113 = property on="All Signals" class="WFChart (strict)"("LegNumRows"=w1751) -> ()  [unwired: 2 in, 2 out]
      }
      event "Adjust Scale\nto Mean": Value Change {
        n1114 = event-data() -> ()  [unwired: 7 out]
        n1115 = local read "APD rates cluster"() -> (w1762:T1)
        n1116 = Unbundle By Name(w1762) -> ("APD 1 Rate (Hz)"=w1761:dbl)
        n1117 = Multiply(x=1000.0, y="Above (kHz)") -> (x*y=w1768:dbl)
        n1118 = Multiply(x=1000.0, y="Below (kHz)") -> (x*y=w1766:dbl)
        n1119 = Add(x=w1768, y=w1761) -> (x+y=w1763:dbl)
        n1120 = Subtract(x=w1761, y=w1766) -> (x-y=w1764:dbl)
        n1121 = property on="APD Chart" class="WFChart (strict)"("YScale.Minimum"=w1764) -> ()  [unwired: 2 in, 2 out]
        n1122 = property on="APD Chart" class="WFChart (strict)"("YScale.Maximum"=w1763) -> ()  [unwired: 2 in, 2 out]
      }
      event "Phase adj. (AI1)", "+ phase (AI1)", "- phase (AI1)": Value Change {
        n1123 = event-data() -> ()  [unwired: 7 out]
        n1124 = Negate(x="Phase adj. (AI1)") -> (-x=w1780:i16)
        n1125 = Select(t=w1780, s="- phase (AI1)", f="Phase adj. (AI1)") -> (s? t:f=w1779:i16)
        n1126 = xnode "Read/Write Control"("FPGA VI Reference In"=w1772, "Phase count adjustment"=w1779) -> ("FPGA VI Reference Out"=w1778:T41, "error out"=w1777:errorcluster)  [unwired: 2 in]
        n1127 = Or(x="- phase (AI1)", y="+ phase (AI1)") -> (x .or. y?=w1774:bool)
        n1128 = xnode "Read/Write Control"("FPGA VI Reference In"=w1778, "error in"=w1777, "+ phase"=w1774) -> ("error out"=w1773:errorcluster)  [unwired: 1 in, 1 out]
      }
      event "Signals to Plot": Double Click {
        w1792 = u32 9868950 ("Color Box")
        n1129 = event-data() -> ("Row"=w1783:i32)  [unwired: 9 out]
        n1130 = property on="All Signals" class="WFChart (strict)"("Active Plot"=w1783) -> (error out=w1782:errorcluster)  [unwired: 2 in, 1 out]
        n1131 = property on="All Signals" class="WFChart (strict)" props=["Plot", "Plot Color", "Plot", "Visible?"](error in=w1782) -> (error out=w1785:errorcluster, "Plot.Visible?"=w1784:bool)  [unwired: 1 in, 2 out]
        n1132 = Select(t=FALSE ("Plot.Visible"), s=w1784, f=TRUE ("Plot.Visible")) -> (s? t:f=w1787:bool)
        n1133 = property on="All Signals" class="WFChart (strict)"(error in=w1785, "Plot.Visible?"=w1787) -> (error out=w1786:errorcluster)  [unwired: 1 in, 1 out]
        n1134 = property on="All Signals" class="WFChart (strict)"(error in=w1786) -> (error out=w1788:errorcluster, "Plot.Plot Color"=w1789:u32)  [unwired: 1 in, 1 out]
        n1135 = property on="Signals to Plot" class="LstBox (strict)"(error in=w1788, "Active Row"=w1783) -> (error out=w1793:errorcluster)  [unwired: 1 in, 1 out]
        n1136 = Select(t=w1789, s=w1787, f=u32 0) -> (s? t:f=w1794:u32)
        n1137 = property on="Signals to Plot" class="LstBox (strict)"(error in=w1793, "CellFontColor"=w1794, "SelColor"=w1792, "CellBG"=w1792, "CellFontSize"=u32 20 ("Active Row:Cell Font:Size"), "CellFontBold"=TRUE ("Active Row:Cell Font:Bold")) -> ()  [unwired: 1 in, 2 out]
      }
      event "BD 1 Frequency 1 (MHz)", "BD 1 Frequency 2 (MHz)", "BD 1 Frequency 3 (MHz)", "BD 2 Frequency 1 (MHz)", "BD 2 Frequency 2 (MHz)", "BD 2 Frequency 3 (MHz)", "Trap Delta (MHz)", "Update all trap values": Value Change {
        # "This is so you can set trap frequencies\nvia local variables and then update\nall at once"
        n1138 = event-data() -> ("CtlRef"=w1802:refnum<vi>)  [unwired: 6 out]
        n1139 = control-ref of="Trap Delta (MHz)"() -> (w1801:refnum<vi>)
        n1140 = Equal?(x=w1801, y=w1802) -> (x = y?=w1800:bool)
        n1141 = local write "Update all trap values"(FALSE ("Update all trap values")) -> ()
        n1142 = case shown="False" "Oscillate Set 1" {
          tunnel: w1800 -> [w1816 _]
          tunnel: w1798 -> [w1814 _]
          frame False {
            n1143 = local read "BD 1 Frequency 2 (MHz)"() -> (w1812:dbl)
            n1144 = case shown="False" "Symmetric?" {
              tunnel: "Trap Delta (MHz)" -> [w1838 w1845]
              tunnel: [w1839 w1843] -> w1804
              tunnel: [w1837 w1840] -> w1806
              tunnel: w1812 -> [w1839 _]
              frame False {
                n1145 = Subtract(x=w1839, y=w1838) -> (x-y=w1837:dbl)
              }
              frame True {
                w1842 = 75
                n1146 = Divide(x=w1845, y=2.0) -> (x/y=w1841:dbl)
                n1147 = Add(x=w1841, y=w1842) -> (x+y=w1843:dbl)
                n1148 = Subtract(x=w1842, y=w1841) -> (x-y=w1840:dbl)
              }
            }
            n1149 = local read "BD 1 Frequency 1 (MHz)"() -> (w1807:dbl)
            n1150 = Not(x="Symmetric?") -> (.not. x?=w1810:bool)
            n1151 = And(x=w1810, y="move Con X?") -> (x .and. y?=w1808:bool)
            n1152 = Subtract(x=w1807, y=w1806) -> (x-y=w1805:dbl)
            n1153 = Select(t=w1806, s=w1816, f=w1807) -> (s? t:f=w1815:dbl)
            n1154 = local read "Y RF Frequency Limits (MHz)"() -> (w1817:T23)
            n1155 = case shown="True" w1808 {
              tunnel: w1805 -> [_ w1836]
              frame False {
              }
              frame True {
                n1156 = property on="AOM X Cal (nm/MHz)" class="DigNum (strict)"() -> ("Value"=w1835:dbl)  [unwired: 2 in, 2 out]
                n1157 = property on="MCL Step Position Ratio" class="DigNum (strict)"() -> ("Value"=w1829:dbl)  [unwired: 2 in, 2 out]
                n1158 = Compound Arithmetic op=MULTIPLY(w1836, w1835, w1829) -> (w1834:dbl)
                n1159 = property on="MCL X Cal (nm/V)" class="DigNum (strict)"() -> ("Value"=w1833:dbl)  [unwired: 2 in, 2 out]
                n1160 = Divide(x=w1834, y=w1833) -> (x/y=w1832:dbl)
                n1161 = property on="AO2" class="Slide (strict)"() -> ("Value"=w1831:dbl)  [unwired: 2 in, 2 out]
                n1162 = Add(x=w1832, y=w1831) -> (x+y=w1830:dbl)
                n1163 = property on="AO2" class="Slide (strict)"("Val(Sgnl)"=w1830) -> ()  [unwired: 2 in, 2 out]
              }
            }
            n1164 = local read "X RF Frequency Limits (MHz)"() -> (w1818:T23)
            n1165 = local write "BD 1 Frequency 1 (MHz)"(w1815) -> ()
            n1166 = local read "BD 1 Frequency 3 (MHz)"() -> (w1827:dbl)
            n1167 = local read "BD 2 Frequency 1 (MHz)"() -> (w1821:dbl)
            n1168 = local read "BD 2 Frequency 2 (MHz)"() -> (w1820:dbl)
            n1169 = local read "BD 2 Frequency 3 (MHz)"() -> (w1828:dbl)
            n1170 = call "set RF board frequency - interlace.vi"("Board 2 Frequency Limits"=w1817, "Board 1 Frequency Limits"=w1818, "FPGA VI Reference In"=w1814, "Board 2 Frequency 3 (MHz)"=w1828, "Board 1 Frequency 3 (MHz)"=w1827, "Board 2 Frequency 2 (MHz)"=w1820, "Board 2 Frequency 1 (MHz)"=w1821, "Board 1 Frequency 2 (MHz)"=w1804, "Board 1 Frequency 1  (MHz)"=w1815) -> ()  [unwired: 1 in, 2 out]
            n1171 = Subtract(x=w1821, y=w1820) -> (x-y=w1825:dbl)
            n1172 = local write "BD 1 Frequency 2 (MHz)"(w1804) -> ()
            n1173 = Subtract(x=w1815, y=w1804) -> (x-y=w1826:dbl)
            n1174 = Square(x=w1825) -> (x^2=w1823:dbl)
            n1175 = Square(x=w1826) -> (x^2=w1824:dbl)
            n1176 = Add(x=w1824, y=w1823) -> (x+y=w1822:dbl)
            n1177 = Square Root(x=w1822) -> (sqrt(x)=w1819:dbl)
            n1178 = property on="Initial delta (MHz)" class="DigNum (strict)"("Val(Sgnl)"=w1819) -> ()  [unwired: 2 in, 2 out]
            n1179 = local write "Trap Delta (MHz)"(w1819) -> ()
          }
          frame True {
          }
        }
      }
      event "manual raster set": Value Change {
        n1180 = event-data() -> ()  [unwired: 7 out]
        n1181 = flat-sequence {
          frame #0 {
            n1182 = Replace Array Subset(array=u32[] [0] ("Index Values"), new element="manual raster set", index=0) -> (w1846:u32[])
            n1183 = property on="Saved AOD Raster Scan Parameter Sets" class="Arr (strict)"("Index Values"=w1846) -> ()  [unwired: 2 in, 2 out]
          }
          frame #1 {
            n1184 = property on="Load parameters" class="Bool (strict)"("Val(Sgnl)"=TRUE ("Value (Signaling)")) -> ()  [unwired: 2 in, 2 out]
          }
        }
      }
      event "Round T1 X": Value Change {
        n1185 = event-data() -> ()  [unwired: 7 out]
        n1186 = local read "BD 1 Frequency 1 (MHz)"() -> (w1853:dbl)
        n1187 = Round To Nearest(number=w1853) -> (nearest integer value=w1852:dbl)
        n1188 = property on="BD 1 Frequency 1 (MHz)" class="DigNum (strict)"("Val(Sgnl)"=w1852) -> ()  [unwired: 2 in, 2 out]
      }
      event "Round T2 X": Value Change {
        n1189 = event-data() -> ()  [unwired: 7 out]
        n1190 = local read "BD 1 Frequency 2 (MHz)"() -> (w1855:dbl)
        n1191 = Round To Nearest(number=w1855) -> (nearest integer value=w1854:dbl)
        n1192 = property on="BD 1 Frequency 2 (MHz)" class="DigNum (strict)"("Val(Sgnl)"=w1854) -> ()  [unwired: 2 in, 2 out]
      }
      event "Stop All": Value Change {
        n1193 = event-data() -> ()  [unwired: 7 out]
        n1194 = flat-sequence {
          tunnel: [w1861] -> w1859
          tunnel: [w1864] -> w1857
          tunnel: w1859 -> [w1864]
          tunnel: [TRUE] -> w1858
          frame #0 {
            n1195 = local read "Visa resource for valves"() -> (w1860:refnum<visa-resource-name>)
            n1196 = call "hamilton_controller.vi"("VISA resource name in"=w1860, "action"=T42."DISCONNECT") -> ("error out"=w1861:errorcluster)  [unwired: 8 in, 1 out]
          }
          frame #1 {
          }
        }
      }
      event "Delayed Interlace Start": Value Change {
        n1197 = event-data() -> ()  [unwired: 7 out]
        n1198 = flat-sequence {
          frame #0 {
            n1199 = Multiply(x="Delay to Interlace (s)", y=1000.0) -> (x*y=w1866:dbl)
            n1200 = Wait (ms)(milliseconds to wait=w1866) -> ()  [unwired: 1 out]
          }
          frame #1 {
            n1201 = property on="Laser interlacing mode" class="RadioBtnsControl (strict)"("Val(Sgnl)"=enum32{"Laser ON", "Laser OFF", "Interlace"}."Interlace" ("Value (Signaling)")) -> ()  [unwired: 2 in, 2 out]
          }
        }
      }
      event "BD 1 Amplitude 1 (%)", "BD 1 Amplitude 2 (%)", "BD 1 Amplitude 3 (%)", "BD 2 Amplitude 1 (%)", "BD 2 Amplitude 2 (%)", "BD 2 Amplitude 3 (%)", "Trap 1 ON", "Trap 2 ON", "Trap 3 ON", "Feedback On/Off", "All FB On/Off": Value Change {
        w1891 = i16 1 ("f")
        n1202 = event-data() -> ()  [unwired: 7 out]
        n1203 = local write "Trap 1 (ON/OFF)"("Trap 1 ON") -> ()
        n1204 = local write "Trap 2 (ON/OFF)"("Trap 2 ON") -> ()
        n1205 = Boolean To (0,1)(Boolean="Trap 3 ON") -> (0, 1=w1892:i16)
        n1206 = Boolean To (0,1)(Boolean="Trap 1 ON") -> (0, 1=w1893:i16)
        n1207 = Boolean To (0,1)(Boolean="Trap 2 ON") -> (0, 1=w1894:i16)
        n1208 = Select(t=w1894, s="Trap ON/OFF X or Y Amp?", f=w1891) -> (s? t:f=w1889:i16)
        n1209 = Select(t=w1893, s="Trap ON/OFF X or Y Amp?", f=w1891) -> (s? t:f=w1890:i16)
        n1210 = Select(t=w1892, s="Trap ON/OFF X or Y Amp?", f=w1891) -> (s? t:f=w1888:i16)
        n1211 = Select(t=w1891, s="Trap ON/OFF X or Y Amp?", f=w1894) -> (s? t:f=w1886:i16)
        n1212 = Select(t=w1891, s="Trap ON/OFF X or Y Amp?", f=w1893) -> (s? t:f=w1887:i16)
        n1213 = Select(t=w1891, s="Trap ON/OFF X or Y Amp?", f=w1892) -> (s? t:f=w1885:i16)
        n1214 = And(x="All FB On/Off", y="Feedback On/Off") -> (x .and. y?=w1883:cluster{"Set 1":bool, "Set 2":bool})
        n1215 = local read "BD 1 Amplitude 1 (%)"() -> (w1901:dbl)
        n1216 = local read "BD 1 Amplitude 2 (%)"() -> (w1900:dbl)
        n1217 = local read "BD 1 Amplitude 3 (%)"() -> (w1899:dbl)
        n1218 = Unbundle By Name(w1883) -> ("Set 1"=w1878:bool, "Set 2"=w1875:bool)
        n1219 = local read "Y RF Amplitude Limits (%)"() -> (w1871:T23)
        n1220 = local read "X RF Amplitude Limits (%)"() -> (w1872:T23)
        n1221 = local read "BD 2 Amplitude 1 (%)"() -> (w1902:dbl)
        n1222 = local read "BD 2 Amplitude 2 (%)"() -> (w1903:dbl)
        n1223 = local read "BD 2 Amplitude 3 (%)"() -> (w1904:dbl)
        n1224 = And(x="Trap 2 ON", y=w1875) -> (x .and. y?=w1873:bool)
        n1225 = And(x="Trap 1 ON", y=w1878) -> (x .and. y?=w1876:bool)
        n1226 = Multiply(x=w1890, y=w1901) -> (x*y=w1898:dbl)
        n1227 = Multiply(x=w1900, y=w1889) -> (x*y=w1896:dbl)
        n1228 = Multiply(x=w1899, y=w1888) -> (x*y=w1897:dbl)
        n1229 = Multiply(x=w1902, y=w1887) -> (x*y=w1905:dbl)
        n1230 = Multiply(x=w1903, y=w1886) -> (x*y=w1906:dbl)
        n1231 = Multiply(x=w1904, y=w1885) -> (x*y=w1907:dbl)
        n1232 = call "set RF board amplitude - interlace.vi"("Board 2 Amplitude Limits"=w1871, "Board 1 Amplitude Limits"=w1872, "FPGA VI Reference In"=w1870, "Board 2 Amplitude 3 (%)"=w1907, "Board 1 Amplitude 3 (%)"=w1897, "Board 2 Amplitude 2 (%)"=w1906, "Board 2 Amplitude 1 (%)"=w1905, "Board 1 Amplitude 2 (%)"=w1896, "Board 1 Amplitude 1 (%)"=w1898) -> ("error out"=w1880:errorcluster, "FPGA VI Reference Out"=w1881:T41)  [unwired: 1 in]
        n1233 = xnode "Read/Write Control"("FPGA VI Reference In"=w1881, "error in"=w1880, "FB On/Off Set 1"=w1876, "FB On/Off Set 2"=w1873) -> ("error out"=w1879:errorcluster)  [unwired: 1 out]
      }
      event "Load parameters": Value Change {
        n1234 = event-data() -> ()  [unwired: 7 out]
        n1235 = property on="Saved AOD Raster Scan Parameter Sets" class="Arr (strict)"() -> ("Index Values"=w1918:u32[])  [unwired: 2 in, 2 out]
        n1236 = Index Array(array=w1918, index=0) -> (element=w1915:u32)
        n1237 = local write "Load parameters"(FALSE ("Load parameters")) -> ()
        n1238 = Index Array(array="Saved AOD Raster Scan Parameter Sets", index=w1915) -> (element=w1914:T46)
        n1239 = Unbundle By Name(w1914) -> ("Scan Range AOD (nm) 2"=w1913:dbl, "Step Size AOD (nm) 2"=w1912:dbl, "Scan Speed AOD (nm/s) 2"=w1911:dbl, "Number of scans (AOD) 2"=w1910:u16)
        n1240 = flat-sequence {
          tunnel: w1913 -> [w1921]
          tunnel: w1912 -> [w1920]
          tunnel: w1911 -> [w1919]
          tunnel: w1910 -> [w1922]
          frame #0 {
            n1241 = local write "Scan Speed (nm/s)"(w1919) -> ()
            n1242 = local write "Scan Range (nm)"(w1921) -> ()
            n1243 = local write "Step Size (nm)"(w1920) -> ()
          }
          frame #1 {
            n1244 = property on="Number of F/B Scans (AOD)" class="DigNum (strict)"("Val(Sgnl)"=w1922) -> ()  [unwired: 2 in, 2 out]
          }
        }
      }
      event "Trap 1 (ON/OFF)", "Trap 2 (ON/OFF)": Value Change {
        n1245 = event-data() -> ()  [unwired: 7 out]
        n1246 = flat-sequence {
          tunnel: [w1932] -> w1927
          tunnel: w1927 -> [w1947]
          tunnel: [w1933] -> w1923
          frame #0 {
            n1247 = local read "Trap 1 ON"() -> (w1932:bool)
          }
          frame #1 {
            n1248 = Exclusive Or(1:w1947, 2:"Trap 1 (ON/OFF)") -> (0:w1940:bool)
            n1249 = Select(t="on", s="Trap 2 (ON/OFF)", f="off") -> (s? t:f=w1939:string)
            n1250 = Select(t="on", s="Trap 1 (ON/OFF)", f="off") -> (s? t:f=w1935:string)
            n1251 = Build Array("trap 1 ", w1935) -> (w1934:string[])
            n1252 = Build Array("trap 2 " ("f"), w1939) -> (w1937:string[])
            n1253 = Select(t=w1934, s=w1940, f=w1937) -> (s? t:f=w1933:string[])
            n1254 = property on="Trap 1 ON" class="Bool (strict)"("Val(Sgnl)"="Trap 1 (ON/OFF)") -> ()  [unwired: 2 in, 2 out]
            n1255 = property on="Trap 2 ON" class="Bool (strict)"("Val(Sgnl)"="Trap 2 (ON/OFF)") -> ()  [unwired: 2 in, 2 out]
          }
        }
        n1256 = local read "Saving..."() -> (w1926:bool)
        n1257 = local read "Save Event Log?"() -> (w1925:bool)
        n1258 = And(x=w1926, y=w1925) -> (x .and. y?=w1924:bool)
        n1259 = case shown="True" w1924 {
          tunnel: w1923 -> [_ w1931]
          frame False {
          }
          frame True {
            n1260 = local read "Time (s)"() -> (w1928:dbl)
            n1261 = local read "log file ref"() -> (w1930:refnum<file>)
            n1262 = Concatenate Strings(w1931) -> (w1929:string)
            n1263 = call "write to event log.vi"("log file ref"=w1930, "time"=w1928, "input string"=w1929) -> ()  [unwired: 8 in]
          }
        }
      }
      event "DIO count 1 (ticks)", "DIO count 2 (ticks)", "DIO count 3 (ticks)", "Interlace", "Number Interlace Sets", "Not-Interlacing Set", "BD 1 Delay (ticks)", "BD 2 Delay (Ticks)", "Next trap write delay (ticks)", "XY phase ext loop method", "Amp switch delay 2", "BD 2 Delay (Ticks) 2", "BD 1 Delay (ticks) 2": Value Change {
        n1264 = event-data() -> ()  [unwired: 7 out]
        n1265 = To Unsigned Byte Integer(number="Not-Interlacing Set") -> (unsigned 8bit integer=w1948:u8)
        n1266 = Add(x=u8 1 ("y"), y=w1948) -> (x+y=w1957:u8)
        n1267 = local read "DIO count 1 (ticks)"() -> (w1964:u16)
        n1268 = local read "DIO count 2 (ticks)"() -> (w1963:u16)
        n1269 = local read "DIO count 3 (ticks)"() -> (w1962:u16)
        n1270 = xnode "Read/Write Control"("FPGA VI Reference In"=w1950, "DIO count 1 (ticks)"=w1964, "DIO count 2 (ticks)"=w1963, "DIO count 3 (ticks)"=w1962, "Interlace ON/OFF"="Interlace", "Number Interlace Cycles"="Number Interlace Sets", "Interlace Off Parameters"=w1957, "BD 1 Delay (ticks)"="BD 1 Delay (ticks)", "BD 2 Delay (Ticks)"="BD 2 Delay (Ticks)", "Next trap write delay (ticks)"="Next trap write delay (ticks)") -> ("error out"=w1966:errorcluster)  [unwired: 1 in, 1 out]
        n1271 = Build Array(w1964, w1963, w1962) -> (w1956:u16[])
        n1272 = Split 1D Array(array=w1956, index="Number Interlace Sets") -> (first subarray=w1965:u16[])  [unwired: 1 out]
        n1273 = Index Array(array=w1956, index=w1948) -> (element=w1955:u16)
        n1274 = Add Array Elements(numeric array=w1965) -> (sum=w1959:u16)
        n1275 = Select(t=w1959, s="Interlace", f=w1955) -> (s? t:f=→"Total Counts (ticks)":u16)
      }
      event "Reset Feedback": Value Change {
        n1276 = event-data() -> ()  [unwired: 7 out]
        n1277 = Unbundle By Name("Reset Feedback") -> ("Set 1"=w1970:bool, "Set 2"=w1969:bool)
        n1278 = xnode "Read/Write Control"("FPGA VI Reference In"=w1967, "FB Reset Set 1"=w1970, "FB Reset Set 2"=w1969) -> ("error out"=w1968:errorcluster)  [unwired: 1 in, 1 out]
      }
      event "Trap intensity output range", "Trap Intensity PID Gains": Value Change {
        n1279 = event-data() -> ()  [unwired: 7 out]
        n1280 = xnode "Read/Write Control"("FPGA VI Reference In"=w1974, "FB Gains"="Trap Intensity PID Gains", "FB output range"="Trap intensity output range") -> ("error out"=w1975:errorcluster)  [unwired: 1 in, 1 out]
      }
      event "AI2 to Setpoint", "Setpoints (V)": Value Change {
        n1281 = event-data() -> ()  [unwired: 7 out]
        n1282 = xnode "Read/Write Control"("FPGA VI Reference In"=w1976) -> ("FPGA VI Reference Out"=w1979:T41, "error out"=w1978:errorcluster, "AI2 Y Sum Set 1"=w1986:i16, "AI2 Y Sum Set 2"=w1985:i16)  [unwired: 1 in]
        n1283 = Cluster To Array(cluster="AI2 to Setpoint") -> (array=w1989:bool[])
        n1284 = local read "AI2 (V)"() -> (w1987:cluster{"Set 1":dbl, "Set 2":dbl})
        n1285 = Or Array Elements(Boolean array=w1989) -> (logical OR=w1990:bool)
        n1286 = Bundle By Name(cluster=w1987, "Set 1"=w1986, "Set 2"=w1985) -> (w1984:cluster{"Set 1":dbl, "Set 2":dbl})
        n1287 = Divide(x=w1984, y=3276.7) -> (x/y=w1983:cluster{"Set 1":dbl, "Set 2":dbl})
        "AI2 (V)" <- w1983
        n1288 = case shown="True" w1990 {
          tunnel: [w1993 w2010] -> w1982
          tunnel: "AI2 to Setpoint" -> [_ w2006]
          tunnel: "Setpoints (V)" -> [w1994 w2009]
          tunnel: w1983 -> [_ w2003]
          frame False {
            n1289 = Multiply(x=3276.7, y=w1994) -> (x*y=w1995:cluster{"Set 1":dbl, "Set 2":dbl})
            n1290 = To Word Integer(number=w1995) -> (16bit integer=w1993:cluster{"Set 1":i16, "Set 2":i16})
          }
          frame True {
            n1291 = Unbundle By Name(w2003) -> ("Set 1"=w2002:dbl, "Set 2"=w2001:dbl)
            n1292 = Unbundle By Name(w2009) -> ("Set 1"=w2008:dbl, "Set 2"=w2007:dbl)
            n1293 = Unbundle By Name(w2006) -> ("Set 1"=w2005:bool, "Set 2"=w2004:bool)
            n1294 = Select(t=w2002, s=w2005, f=w2008) -> (s? t:f=w2000:dbl)
            n1295 = Select(t=w2001, s=w2004, f=w2007) -> (s? t:f=w1999:dbl)
            n1296 = Bundle By Name(cluster=w2009, "Set 1"=w2000, "Set 2"=w1999) -> (w1997:cluster{"Set 1":dbl, "Set 2":dbl})
            n1297 = local write "Setpoints (V)"(w1997) -> ()
            n1298 = Multiply(x=3276.7, y=w1997) -> (x*y=w1998:cluster{"Set 1":dbl, "Set 2":dbl})
            n1299 = To Word Integer(number=w1998) -> (16bit integer=w2010:cluster{"Set 1":i16, "Set 2":i16})
          }
        }
        n1300 = Unbundle By Name(w1982) -> ("Set 1"=w1981:i16, "Set 2"=w1980:i16)
        n1301 = xnode "Read/Write Control"("FPGA VI Reference In"=w1979, "error in"=w1978, "FB Setpoint Set 1"=w1981, "FB Setpoint Set 2"=w1980) -> ("error out"=w1977:errorcluster)  [unwired: 1 out]
      }
      event "+ phase (GI)", "- phase (GI)", "+ phase (GI) 2", "- phase (GI) 2", "+ phase (RI)", "- phase (RI)", "+ phase (Green FB)", "- phase (Green FB)", "- phase (BI AO)", "+ phase (BI AO)", "- phase (BI DO)", "+ phase (BI DO)": Value Change {
        n1302 = event-data() -> ()  [unwired: 7 out]
        n1303 = Or(x="+ phase (GI)", y="- phase (GI)") -> (x .or. y?=w2046:bool)
        n1304 = Negate(x="Phase adj. (GI)") -> (-x=w2051:i16)
        n1305 = Select(t=w2051, s="+ phase (GI)", f="Phase adj. (GI)") -> (s? t:f=w2050:i16)
        n1306 = Or(x="+ phase (GI) 2", y="- phase (GI) 2") -> (x .or. y?=w2037:bool)
        n1307 = Negate(x="Phase adj. (GI) 2") -> (-x=w2042:i16)
        n1308 = Select(t=w2042, s="+ phase (GI) 2", f="Phase adj. (GI) 2") -> (s? t:f=w2038:i16)
        n1309 = Negate(x="Phase adj. (RI)") -> (-x=w2036:i16)
        n1310 = Or(x="+ phase (RI)", y="- phase (RI)") -> (x .or. y?=w2032:bool)
        n1311 = Select(t=w2036, s="+ phase (RI)", f="Phase adj. (RI)") -> (s? t:f=w2031:i16)
        n1312 = Or(x="+ phase (Green FB)", y="- phase (Green FB)") -> (x .or. y?=w2025:bool)
        n1313 = Negate(x="Phase adj. (Green FB)") -> (-x=w2030:i16)
        n1314 = Select(t=w2030, s="+ phase (Green FB)", f="Phase adj. (Green FB)") -> (s? t:f=w2026:i16)
        n1315 = Negate(x="Phase adj. (BI AO)") -> (-x=w2024:i16)
        n1316 = Or(x="+ phase (BI AO)", y="- phase (BI AO)") -> (x .or. y?=w2014:bool)
        n1317 = Select(t=w2024, s="+ phase (BI AO)", f="Phase adj. (BI AO)") -> (s? t:f=w2016:i16)
        n1318 = Negate(x="Phase adj. (BI DO)") -> (-x=w2020:i16)
        n1319 = Or(x="+ phase (BI DO)", y="- phase (BI DO)") -> (x .or. y?=w2013:bool)
        n1320 = Select(t=w2020, s="+ phase (BI DO)", f="Phase adj. (BI DO)") -> (s? t:f=w2015:i16)
        n1321 = xnode "Read/Write Control"("FPGA VI Reference In"=w2012, "Phase count adjustment (GI)"=w2050, "Phase count adjustment (GI) 2"=w2038, "Phase count adjustment (RI)"=w2031, "Phase count adjustment (Green FB)"=w2026, "Phase count adjustment (BI AO)"=w2016, "Phase count adjustment (BI D)"=w2015) -> ("FPGA VI Reference Out"=w2048:T41, "error out"=w2049:errorcluster)  [unwired: 1 in]
        n1322 = xnode "Read/Write Control"("FPGA VI Reference In"=w2048, "error in"=w2049, "+ phase (GI)"=w2046, "+ phase (GI) 2"=w2037, "+ phase (RI)"=w2032, "+ phase (Green FB)"=w2025, "+ phase (BI AO)"=w2014, "+ phase (BI D)"=w2013) -> ("error out"=w2047:errorcluster)  [unwired: 1 out]